vi "01 Dryer_Performance_SM.vi"() -> ()   [LabVIEW 2012] (continued)
                  tunnel: w1015 -> [w1034 _]
                  tunnel: [w1025 w1043] -> w1014
                  tunnel: [w1024 w1037] -> w1013
                  tunnel: w1012 -> [_ w1041]
                  tunnel: w1011 -> [_ w1040]
                  frame False {
                    n446 = call "AG34980A Initiate.vi"("VISA resource name"=w1036, "error in (no error)"=w1035) -> ("VISA resource name out"=w1032:refnum<visa-resource-name>, "error out"=w1033:errorcluster)  [unwired: 12 in]
                    n447 = call "AG34980A Fetch.vi"("VISA resource name"=w1032, "Numbers Only (T:On)"=TRUE, "error in (no error)"=w1033, "Byte Count (1024 bytes)"=5000) -> ("VISA resource name out"=w1021:refnum<visa-resource-name>, "Output Data (Numbers Only)"=w1027:dbl[], "error out"=w1023:errorcluster)  [unwired: 7 in, 2 out]
                    n448 = call "AG34980A Error Query (Multiple).vi"("VISA resource name"=w1021, "error in (no error)"=w1023) -> ("Error Message"=→"Error Message 2":string, "error out"=w1022:errorcluster)  [unwired: 10 in, 2 out]
                    n449 = Search 1D Array(1D array=w1034, element="Chamber Temp" ("Label")) -> (index of element=w1029:i32)  [unwired: 1 in]
                    n450 = Search 1D Array(1D array=w1034, element="Chamber RH" ("Label")) -> (index of element=w1030:i32)  [unwired: 1 in]
                    n451 = Index Array(array=w1027, index=w1029) -> (element=w1024:dbl)
                    n452 = Index Array(array=w1027, index=w1030) -> (element=w1025:dbl)
                  }
                  frame True {
                    n453 = local read "CDAQ Tasks"() -> (w1044:refnum<k21>[])
                    n454 = call "03 cDAQ Chan Tester.vi"("Tasks In"=w1044, "error in (no error)"=w1039, "Mode"=T18."Gather DATA") -> ("error out"=w1038:errorcluster, "CDAQ Data Out"=w1046:dbl[])  [unwired: 6 in, 1 out]
                    n455 = Decimal String To Number(string=w1041) -> (number=w1045:i32)  [unwired: 2 in, 1 out]
                    n456 = Decimal String To Number(string=w1040) -> (number=w1042:i32)  [unwired: 2 in, 1 out]
                    n457 = Index Array(array=w1046, index #1=w1045, index #2=w1042) -> (element #1=w1043:dbl, element #2=w1037:dbl)
                  }
                }
              }
              frame True {
                n458 = global read "Global Test Variables DPT.vi" "Globals for Dryer Performance Test"() -> (w1052:T9)
                n459 = Unbundle By Name(w1052) -> ("Test Setup.RH-IP"=w1053:string)
                n460 = call "Newport ITX-D3N.vi"("error in (no error)"=w1055, "Machine"=w1053) -> ("error out"=w1054:errorcluster, "[Temp (F), RH]"=w1051:dbl[])  [unwired: 8 in]
                n461 = Array To Cluster(array=w1051) -> (cluster=w1050:T26)
                n462 = Unbundle(w1050) -> ("[Temp (F), RH][0]"=w1049:dbl, "[Temp (F), RH][1]"=w1048:dbl)
              }
            }
            n463 = Number To Fractional String(number=w989, precision (6)=i16 1) -> (F-format string=w988:string)  [unwired: 2 in]
            n464 = Number To Fractional String(number=w986, precision (6)=i16 1) -> (F-format string=w985:string)  [unwired: 2 in]
            n465 = local read "2015?"() -> (w981:bool)
            n466 = Build Array("Ambient Temp", "Ambient RH") -> (w996:string[])
            n467 = Build Array(w985, w988) -> (w995:string[])
            n468 = Build Array(w996, w995) -> (w1004:string[][])
            n469 = call "Worksheet DOE Audit.vi"() -> ("DOE Data Out"=w991:T23)  [unwired: 8 in, 2 out]
            n470 = Bundle By Name(cluster=w991, "Ambinet Temp"=w985, "Ambinet RH"=w988) -> (w992:T23)
            n471 = Transpose 2D Array(2D array=w1004) -> (transposed array=w1003:string[][])
            n472 = Build Array (concatenate)(w1006, w1003) -> (w1005:string[][])
            n473 = Bundle By Name(cluster=w1008, "Start Header Data"=w1005) -> (w1007:T22)
            n474 = call "Worksheet DOE Audit.vi"("Add?"=TRUE, "DOE Data"=w992, "2015?"=w981) -> ()  [unwired: 5 in, 3 out]
          }
          frame True {
          }
        }
        n475 = case shown="Error" w972 {
          tunnel: ["" ("State(s) in Front (\"\")") "Macro: Exit" ("State(s) in Front (\"\")")] -> w978
          tunnel: w977 -> [_ w1060]
          frame No Error {
          }
          frame Error {
            n476 = Concatenate Strings("Error:", w1060) -> (w1062:string)
            n477 = One Button Dialog(message=w1062) -> ()  [unwired: 1 in, 1 out]
          }
        }
        n478 = call <vilib>:"Add State(s) to Queue__jki_lib_state_machine.vi"("State(s) in Front (\"\")"=w978, "State(s) in (\"\")"=w980) -> ("States Out"=w979:string)  [unwired: 13 in]
      }
      frame "Start: Files" {
        # "Preceeded by:\n Dryer Weight setting in Global."
        # "Alter File Init subvi per application to get a dialog box that gives you \nyour data filename."
        n479 = global read "Global Test Variables DPT.vi" "Globals for Dryer Performance Test"() -> (w1066:T9)
        n480 = local read "cDAQ"() -> (w1079:bool)
        n481 = Unbundle By Name(w1088) -> ("Start Header Data"=w1085:string[][])
        n482 = case shown="True" w1079 {
          frame False {
          }
          frame True {
            # "Keep CDAQ Buffer Empty"
            n483 = while {
              stop <- w1099 stop-if-true
              n484 = local read "CDAQ Tasks"() -> (w1100:refnum<k21>[])
              n485 = local read "Write to File"() -> (w1099:bool)
              n486 = call "03 cDAQ Chan Tester.vi"("Tasks In"=w1100, "Mode"=T18."Gather DATA") -> ()  [unwired: 7 in, 3 out]
              n487 = Wait (ms)(milliseconds to wait=u32 1000) -> ()  [unwired: 1 out]
            }
          }
        }
        n488 = Unbundle By Name(w1066) -> ("Directories.Work File Directory"=w1065:path)
        "Work File Directory" <- w1065
        n489 = local read "FileVersionInfo Out"() -> (w1080:T5)
        n490 = Unbundle By Name(w1080) -> ("ProductName"=w1095:string, "FileVersion"=w1094:string)
        n491 = local read "Scale Com Port"() -> (w1082:refnum<visa-resource-name>)
        n492 = call "Panel Data_File_Init DPT.vi"("Data File Directory"=w1065, "Test_Title Per TR:"="DPT" ("Test_Title*:"), "Scale Com Port"=w1082, "Test_Type:"=w1095, "Version In:"=w1094, "Supply Voltage:"="Supply Voltage:", "Flow Computer Info Baro,BTUF,u,Z"=w1085, "error in (no error)"=w1081, "File Extension:"="tmp") -> ("FileName"=w1068:path, "Nominal Load  Weight"=w1063:string, "Weights Out"=w1087:T27, "error out"=w1072:errorcluster)  [unwired: 2 in, 1 out]
        "FileName DataLog" <- w1068
        n493 = Bundle By Name(cluster=w1088, "Dryer Load Nominal Weight"=w1063) -> (w1064:T22)
        n494 = Strip Path(path=w1068) -> (name=w1078:string)  [unwired: 1 out]
        "Data Filename" <- w1078
        n495 = Match Pattern(string=w1078, regular expression="\\.") -> (before substring=w1076:string)  [unwired: 1 in, 3 out]
        n496 = Concatenate Strings(w1076, "_DC_AI.csv" ("string")) -> (w1073:string)
        n497 = Unbundle By Name(w1087) -> ("Actual RMC"=w1086:dbl, "Bone Dry Wt(lbs)"=w1084:dbl, "Measured IMC"=w1083:dbl)
        "BDW - Bone Dry Wt(lbs)" <- w1084
        "Wet Clothing Weight" <- w1083
        n498 = Build Path(base path=w1065, name or relative path=w1073) -> (appended path=w1074:path)
        n499 = local write "DC Voltages Filename"(w1074) -> ()
        n500 = Equal?(x=path "", y=w1068) -> (x = y?=w1067:bool)
        n501 = Unbundle By Name(w1072) -> ("status"=w1070:bool)
        n502 = flat-sequence {
          tunnel: w1084 -> [w1105]
          tunnel: w1083 -> [w1104]
          frame #0 {
            n503 = local read "2015?"() -> (w1102:bool)
            n504 = call "Worksheet DOE Audit.vi"() -> ("DOE Data Out"=w1107:T23)  [unwired: 8 in, 2 out]
            n505 = Bundle By Name(cluster=w1107, "Bone Dry Wt"=w1105, "Initial Wt"=w1104) -> (w1106:T23)
            n506 = call "Worksheet DOE Audit.vi"("Add?"=TRUE, "DOE Data"=w1106, "2015?"=w1102) -> ()  [unwired: 5 in, 3 out]
          }
        }
        n507 = local write "RMC%"(w1086) -> ()
        n508 = Or(x=w1067, y=w1070) -> (x .or. y?=w1071:bool)
        n509 = case shown="False" w1071 {
          tunnel: ["" ("State(s) in Front (\"\")") "Macro: Exit" ("State(s) in Front (\"\")")] -> w1089
          tunnel: w1090 -> [_ w1111]
          frame False {
            w1108 = TRUE
            n510 = property on="Write to File" class="Bool (strict)"("Val(Sgnl)"=w1108) -> ()  [unwired: 2 in, 2 out]
            "Write to File" <- w1108
          }
          frame True {
            n511 = Concatenate Strings("Error:", w1111) -> (w1113:string)
            n512 = One Button Dialog(message=w1113) -> ()  [unwired: 1 in, 1 out]
          }
        }
        n513 = call <vilib>:"Add State(s) to Queue__jki_lib_state_machine.vi"("State(s) in Front (\"\")"=w1089, "State(s) in (\"\")"=w1097) -> ("States Out"=w1096:string)  [unwired: 13 in]
      }
      frame "Get Offset Coeff" {
        # "w45 is the weight shift 45 seconds into the test.  The dryer scales have up to a 40 second averaging filter.\nAt 45 seconds after the dryer starts, take the weight adjusted for temp, and subtract from initial conditions.\nThis shift is correlated to the error at the end, depending on the load size."
        # "The conversion of weight to real weight:\n\nBase on load weight (first col).\nCoef of initial weight shift (second col.)\nOffset based on average error seen.  3rd col\nVolume used for temp calculations 4th col."
        n514 = global read "Global Test Variables DPT.vi" "Globals for Dryer Performance Test"() -> (w1116:T9)
        n515 = Unbundle By Name(w1133) -> ("Dryer Load Nominal Weight"=w1131:string)
        n516 = Decimal String To Number(string=w1131, default (0L)=0.0) -> (number=w1117:dbl)  [unwired: 1 in, 1 out]
        n517 = Unbundle By Name(w1116) -> ("Test Setup.T45_Coeff."=w1115:dbl, "Test Setup.Weight Offset"=w1114:dbl)
        n518 = In Range and Coerce(upper limit=3.0, x=w1117, lower limit=0.0) -> (In Range?=w1120:bool)  [unwired: 1 out]
        n519 = In Range and Coerce(upper limit=20.0, x=w1117, lower limit=4.0) -> (In Range?=w1122:bool)  [unwired: 1 out]
        n520 = In Range and Coerce(upper limit=4.0, x=w1117, lower limit=3.0) -> (In Range?=w1121:bool)  [unwired: 1 out]
        n521 = Build Array(w1120, w1121, w1122) -> (w1119:bool[])
        n522 = Boolean Array To Number(Boolean array=w1119) -> (number=w1118:u32)
        n523 = disable-structure shown="Disabled" {
          disable-tunnel: [w1139 w1147] -> w1134
          disable-tunnel: [w1138 w1146] -> w1129
          disable-tunnel: w1118 -> [w1137 _]
          disable-tunnel: w1115 -> [_ w1147]
          disable-tunnel: w1114 -> [_ w1146]
          frame Disabled {
            n524 = case shown="2" w1137 {
              tunnel: [0.0 ("Measured IMC") -1.3651 ("Measured IMC") -1.0373 ("Measured IMC")] -> w1139
              tunnel: [0.055 ("Offset") 0.0378 ("Offset") 0.0348 ("Offset")] -> w1138
              frame 0, Default {
              }
              frame 2 {
                # "4 lb load"
              }
              frame 1 {
              }
            }
          }
          frame Enabled {
          }
        }
        "Init Offset Coeff" <- w1134
        "Offset" <- w1129
        n525 = call <vilib>:"Add State(s) to Queue__jki_lib_state_machine.vi"("State(s) in (\"\")"=w1136) -> ("States Out"=w1135:string)  [unwired: 14 in]
      }
      frame "Start: Time" {
        # "Get stop condition.  Keep reading channels because cdaq gives error if buffer overflows."
        n526 = call "Panel Stop Condition.vi"() -> ("Enable Time Limit Out"=→"Enable Time Limit":bool, "Time Limit(s) Out"=→"Time Limit(s)":dbl, "Enable RMC Limit Out"=→"Enable RMC Limit":bool, "RMC Limit Out"=→"RMC Limit":dbl, "Enable Stop On Power Off Out"=→"Enable Stop On Power Off":bool, "Power Off Time(samples) Out"=→"Power Off Time(samples)":i32, "Power Off Check"=→"Power Off Check":bool[])  [unwired: 9 in]
        n527 = local read "cDAQ"() -> (w1148:bool)
        n528 = case shown="True" w1148 {
          frame False {
          }
          frame True {
            # "Keep CDAQ Buffer Empty"
            n529 = while {
              stop <- w1161 stop-if-true
              n530 = local read "CDAQ Tasks"() -> (w1162:refnum<k21>[])
              n531 = local read "Write to File"() -> (w1161:bool)
              n532 = call "03 cDAQ Chan Tester.vi"("Tasks In"=w1162, "Mode"=T18."Gather DATA") -> ()  [unwired: 7 in, 3 out]
              n533 = Wait (ms)(milliseconds to wait=u32 1000) -> ()  [unwired: 1 out]
            }
          }
        }
        n534 = call <vilib>:"Add State(s) to Queue__jki_lib_state_machine.vi"("State(s) in (\"\")"=w1159) -> ("States Out"=w1158:string)  [unwired: 14 in]
      }
      frame "---------- Data ----------" {
        # "Do not put any code in this frame.\n(It is a separator no-op. You can make a copy of this frame to create a new Data frame)"
        n535 = call <vilib>:"Add State(s) to Queue__jki_lib_state_machine.vi"("State(s) in (\"\")"=w1167) -> ("States Out"=w1166:string)  [unwired: 14 in]
      }
      frame "Data: Initialize" {
        w1168 = ""  # Dryer Load Nominal Weight
        w1169 = ""  # Dryer Type
        w1170 = string[][] []  # Start Header Data
        w1171 = 0.0  # Empty Dryer Cold Weight
        w1172 = "240/120"  # Supply Voltage:
        w1173 = string[] []  # DAQ Label List
        w1174 = ""  # DAQ Chan List
        w1175 = T6 {"Com Agilent"="COM1", "Com Flow Computer"="COM1", "Com Power Meter"="COM1", "Com Power Supply"=""}  # Equipment
        w1176 = path "C:/work/DryerPerformanceTest.ini"  # Config File Path
        w1177 = path "c:/palceholder.csv"  # FileName
        w1179 = errorcluster[] []  # Error Log
        w1180 = T28 {"Current VI Reference"=refnum, "Close Panel on Exit?"=FALSE}  # Core
        # "Config File Name"
        # "Initialize the shift-register data, here.\n(data names are defined by what you wire into the bundle function)"
        n536 = call <vilib>:"Add State(s) to Queue__jki_lib_state_machine.vi"("State(s) in (\"\")"=w1183) -> ("States Out"=w1182:string)  [unwired: 14 in]
        n537 = Bundle("Core"=w1180, "Error Log"=w1179, "FileName"=w1177, "Config File Path"=w1176, "Equipment"=w1175, "DAQ Chan List"=w1174, "DAQ Label List"=w1173, "Supply Voltage:"=w1172, "Empty Dryer Cold Weight"=w1171, "Start Header Data"=w1170, "Dryer Type"=w1169, "Dryer Load Nominal Weight"=w1168) -> (w1181:T22)  [unwired: 1 in]
      }
      frame "Data: Cleanup" {
        # "Cleanup any data and references, here.\n(this is called automatically, by the Macro: Exit)"
        n538 = Unbundle By Name(w1191) -> ("Core.Current VI Reference"=w1190:refnum<vi>, "Equipment.Com Flow Computer"=w1187:refnum<visa-resource-name>, "Equipment"=w1186:T6)
        n539 = flat-sequence {
          tunnel: w1190 -> [w1208]
          tunnel: w1189 -> [w1207]
          tunnel: [w1201] -> w1188
          tunnel: w1187 -> [w1206]
          tunnel: w1185 -> [w1204]
          tunnel: [w1202] -> w1184
          frame #0 {
            w1194 = TRUE ("Finish")
            n540 = Not(x=w1194) -> (.not. x?=w1195:bool)
            n541 = property on="End1_Main" class="Bool (strict)"("Val(Sgnl)"=w1194) -> ()  [unwired: 2 in, 2 out]
            n542 = global write "Nufi Global_ReceivedDataCluster.vi" "Exit Nufi"(w1194) -> ()
            n543 = local write "Start Test"(w1195) -> ()
            "End1_Main" <- w1194
          }
          frame #1 {
            n544 = while {
              stop <- w1200 stop-if-true
              n545 = local read "End2_DAQ"() -> (w1199:bool)
              n546 = local read "End4_Nufi"() -> (w1196:bool)
              n547 = local read "Eng3_Log"() -> (w1198:bool)
              n548 = Compound Arithmetic op=AND(w1196, w1199, w1198) -> (w1200:bool)
              n549 = Wait (ms)(milliseconds to wait=u32 150) -> ()  [unwired: 1 out]
            }
          }
          frame #2 {
            n550 = local read "Use SL9200 Gas Readings?"() -> (w1205:bool)
            n551 = for {
              tunnel: w1204 -> [w1212] mode=indexing
              n552 = VISA Close(VISA resource name=w1212) -> ()  [unwired: 1 in, 1 out]
            }
            n553 = case shown="False" w1205 {
              tunnel: w1206 -> [_ w1214]
              frame False {
              }
              frame True {
                n554 = call "SL9200_Driver_SM.vi"("ComPort"=w1214, "Close Com"=TRUE) -> ()  [unwired: 11 in, 3 out]
              }
            }
            n555 = Close Reference(reference=w1208, error in (no error)=w1207) -> (error out=w1203:errorcluster)
            n556 = case shown="Error" w1203 {
              selector: w1203 -> [w1209 w1210]
              tunnel: [_ "Exit" ("State(s) in Front (\"\")")] -> w1202
              tunnel: [w1209 _] -> w1201
              frame No Error {
              }
              frame Error {
                n557 = call <vilib>:"Simple Error Handler.vi"("error in (no error)"=w1210) -> ()  [unwired: 4 in, 5 out]
              }
            }
          }
        }
        n558 = Cluster To Array(cluster=w1186) -> (array=w1185:refnum<visa-resource-name>[])
        n559 = call <vilib>:"Add State(s) to Queue__jki_lib_state_machine.vi"("State(s) in Front (\"\")"=w1184, "State(s) in (\"\")"=w1193) -> ("States Out"=w1192:string)  [unwired: 13 in]
      }
      frame "---------- UI ----------" {
        # "Do not put any code in this frame.\n(It is a separator no-op. You can make a copy of this frame to create a new UI frame)"
        n560 = call <vilib>:"Add State(s) to Queue__jki_lib_state_machine.vi"("State(s) in (\"\")"=w1218) -> ("States Out"=w1217:string)  [unwired: 14 in]
      }
      frame "UI: Front Panel State" {
        # "Argument"
        # "Set Front Panel Open or Closed\n(Usage: \"UI: Front Panel State >> Open|Close|Minimize\")"
        n561 = Unbundle By Name(w1222) -> ("Core.Current VI Reference"=w1221:refnum<vi>)
        n562 = case shown="True" "Close when complete" {
          tunnel: w1224 -> [w1227 w1231]
          tunnel: [w1227 w1230] -> w1223
          tunnel: w1221 -> [_ w1229]
          tunnel: w1220 -> [_ w1228]
          frame False {
          }
          frame True {
            n563 = case shown="\"Close\"" w1228 {
              tunnel: w1231 -> [w1234 w1238 w1246]
              tunnel: [w1236 w1241 w1247] -> w1230
              tunnel: w1229 -> [w1235 w1237 w1244]
              frame "Open", Default {
                n564 = invoke class="VI" method="FP.Open"(reference=w1235, error in=w1234, "Activate"=TRUE, "State"=T21."Maximized") -> (error out=w1236:errorcluster)  [unwired: 1 in, 4 out]
              }
              frame "Minimize" {
                n565 = invoke class="VI" method="FP.Open"(reference=w1237, error in=w1238, "Activate"=TRUE, "State"=T21."Minimized") -> (error out=w1241:errorcluster)  [unwired: 1 in, 4 out]
              }
              frame "Close" {
                n566 = property class="VI"(reference=w1244, error in=w1246) -> (reference out=w1243:refnum<vi>, error out=w1245:errorcluster, "Front Panel.Open"=w1242:bool)
                n567 = case shown="True" w1242 {
                  tunnel: [w1248 w1251] -> w1247
                  tunnel: w1245 -> [w1248 w1250]
                  tunnel: w1243 -> [_ w1249]
                  frame False {
                  }
                  frame True {
                    n568 = invoke class="VI" method="FP.Close"(reference=w1249, error in=w1250) -> (error out=w1251:errorcluster)  [unwired: 1 in, 2 out]
                  }
                }
              }
            }
          }
        }
        n569 = call <vilib>:"Add State(s) to Queue__jki_lib_state_machine.vi"("State(s) in (\"\")"=w1226) -> ("States Out"=w1225:string)  [unwired: 14 in]
      }
      frame "-------Config File------" {
        # "Do not put any code in this frame.\n(It is a separator no-op. You can make a copy of this frame to create a new Data frame)"
        n570 = call <vilib>:"Add State(s) to Queue__jki_lib_state_machine.vi"("State(s) in (\"\")"=w1255) -> ("States Out"=w1254:string)  [unwired: 14 in]
      }
      frame "Config: Read" {
        w1264 = FALSE  # Write?
        # "Read Globals from Config File.\n(This file will be customized per application)"
        n571 = Unbundle By Name(w1267) -> ("Config File Path"=w1263:path)
        n572 = call "Global Cluster ReadWrite.vi"("Write?"=w1264, "error in (no error)"=w1266, "configuration file path"=w1263) -> ("error out"=w1265:errorcluster, "Test Config Out"=w1257:T9)  [unwired: 7 in]
        n573 = global write "Global Test Variables DPT.vi" "Globals for Dryer Performance Test"(w1257) -> ()
        n574 = local write "Globals for Dryer Performance Test"(w1257) -> ()
        n575 = Unbundle By Name(w1257) -> ("Test Setup.Scale Com"=w1262:dbl, "Test Setup.W. Samps"=w1259:i32, "Test Setup.Smoothing"=→"Use Smoothing":bool, "Test Setup.CDAQ"=→"cDAQ":bool)
        n576 = To Unsigned Byte Integer(number=w1262) -> (unsigned 8bit integer=w1261:u8)
        n577 = call "Com Chan Type Conversion.vi"("Com Chan"=w1261) -> ("VISA resource name"=→"Scale Com Port":refnum<visa-resource-name>)  [unwired: 11 in, 3 out]
        n578 = call <vilib>:"Add State(s) to Queue__jki_lib_state_machine.vi"("State(s) in (\"\")"=w1269) -> ("States Out"=w1268:string)  [unwired: 14 in]
        n579 = local write "W.Samps"(w1259) -> ()
      }
      frame "Config: Write" {
        # "Write Globals to Config File.\n(This file will be customized per application)"
        n580 = Unbundle By Name(w1275) -> ("Config File Path"=w1274:path)
        n581 = global read "Global Test Variables DPT.vi" "Globals for Dryer Performance Test"() -> (w1270:T9)
        "Globals for Dryer Performance Test" <- w1270
        n582 = call "Global Cluster ReadWrite.vi"("Write?"=TRUE, "error in (no error)"=w1273, "configuration file path"=w1274, "Test Config In"=w1270) -> ("error out"=w1272:errorcluster)  [unwired: 6 in, 1 out]
        n583 = call <vilib>:"Add State(s) to Queue__jki_lib_state_machine.vi"("State(s) in (\"\")"=w1277) -> ("States Out"=w1276:string)  [unwired: 14 in]
      }
      frame "---------- Macro ----------" {
        # "Do not put any code in this frame.\n(It is a separator no-op. You can make a copy of this frame to create a new Macro frame)"
        n584 = call <vilib>:"Add State(s) to Queue__jki_lib_state_machine.vi"("State(s) in (\"\")"=w1281) -> ("States Out"=w1280:string)  [unwired: 14 in]
      }
      frame "Macro: Initialize" {
        # "Initialization Macro\n(This is called once, when the VI starts)"
        n585 = call <vilib>:"Add State(s) to Queue__jki_lib_state_machine.vi"("State(s) in Front (\"\")"="Data: Initialize\nInitialize Core Data\nUI: Front Panel State >> Minimize", "State(s) in (\"\")"=w1286) -> ("States Out"=w1285:string)  [unwired: 13 in]
      }
      frame "Macro: Exit" {
        w1296 = "\n"
        w1298 = "Stopping Test" ("String")
        # "Exit Macro\n(This is called once, when the VI exits)"
        n586 = Unbundle By Name(w1300) -> ("Core.Close Panel on Exit?"=w1292:bool)
        n587 = local read "exe?"() -> (w1291:bool)
        n588 = call "String_in_Reference.vi"("String"=w1298) -> ()  [unwired: 18 in, 1 out]
        n589 = local write "Status Message"(w1298) -> ()
        n590 = Compound Arithmetic op=AND(w1292, w1291) -> ()  [unwired: 1 out]
        n591 = Select(t="UI: Front Panel State >> Close", s=FALSE, f="") -> (s? t:f=w1295:string)
        n592 = local write "End Test Button"(FALSE ("End Test")) -> ()
        n593 = Concatenate Strings("Data: Cleanup", w1296, w1295, w1296, "Exit") -> (w1293:string)
        n594 = property on="stop" class="Bool (strict)"("Val(Sgnl)"=TRUE ("Value (Signaling)")) -> ()  [unwired: 2 in, 2 out]
        n595 = call <vilib>:"Add State(s) to Queue__jki_lib_state_machine.vi"("State(s) in Front (\"\")"=w1293, "State(s) in (\"\")"=w1303) -> ("States Out"=w1302:string)  [unwired: 13 in]
      }
      frame "---------- Test ----------" {
        n596 = call <vilib>:"Add State(s) to Queue__jki_lib_state_machine.vi"("State(s) in (\"\")"=w1307) -> ("States Out"=w1306:string)  [unwired: 14 in]
      }
      frame "Test: Main" {
        # "Wait for the test to complete.  Either the button is pressed, or RMC limit is reached, or the time is reached, or the power is off."
        # "Use this as a test to see if the test is complete.  If not, continue to wait."
        n597 = local read "Enable Stop On Power Off"() -> (w1308:bool)
        n598 = local read "Power Off Time(samples)"() -> (w1316:i32)
        n599 = local read "Enable Time Limit"() -> (w1309:bool)
        n600 = local read "Power On One Shot"() -> (w1311:bool)
        n601 = local read "Enable RMC Limit"() -> (w1310:bool)
        n602 = local write "Loggin Data"(TRUE ("Init Complete")) -> ()
        n603 = call "String_in_Reference.vi"("String"="Running, Logging Data...") -> ()  [unwired: 18 in, 1 out]
        n604 = And(x=w1308, y=w1311) -> (x .and. y?=w1317:bool)
        n605 = And(x=w1310, y=w1311) -> (x .and. y?=w1312:bool)
        n606 = case shown="True" w1309 {
          tunnel: [FALSE w1350] -> w1322
          frame False {
          }
          frame True {
            n607 = local read "Start Time (sec)"() -> (w1349:dbl)
            n608 = local read "Time Limit(s)"() -> (w1346:dbl)
            n609 = call "E-Time.vi"() -> ("Elapsed Time (sec)"=w1348:dbl)  [unwired: 9 in, 2 out]
            n610 = Subtract(x=w1348, y=w1349) -> (x-y=w1347:dbl)
            n611 = Greater?(x=w1347, y=w1346) -> (0:w1350:bool)
          }
        }
        n612 = case shown="True" w1312 {
          tunnel: [FALSE w1344] -> w1315
          frame False {
          }
          frame True {
            n613 = local read "RMC Limit"() -> (w1342:dbl)
            n614 = local read "RMC%"() -> (w1343:dbl)
            n615 = Greater?(x=w1342, y=w1343) -> (0:w1344:bool)
          }
        }
        n616 = case shown="True" w1317 {
          selector: w1317 -> [w1329 _]
          tunnel: w1316 -> [_ w1331]
          tunnel: [w1329 w1330] -> w1314
          frame False {
          }
          frame True {
            n617 = disable-structure shown="Enabled" {
              disable-tunnel: w1331 -> [w1338 _]
              disable-tunnel: [w1332 w1340] -> w1330
              frame Disabled {
                n618 = call "Counter.vi"() -> ("Count"=w1339:dbl)  [unwired: 11 in]
                n619 = local read "Power Off Check"() -> (w1335:bool[])
                n620 = Quotient & Remainder(x=w1339, y=w1338) -> (x-y*floor(x/y)=w1337:dbl)  [unwired: 1 out]
                n621 = local read "Power On"() -> (w1336:bool)
                n622 = Replace Array Subset(array=w1335, new element=w1336, index=w1337) -> (w1334:bool[])
                n623 = local write "Power Off Check"(w1334) -> ()
                n624 = Not(x=w1334) -> (.not. x?=w1333:bool[])
                n625 = And Array Elements(Boolean array=w1333) -> (logical AND=w1332:bool)
              }
              frame Enabled {
                n626 = local read "Power Off One Shot"() -> (w1340:bool)
              }
            }
          }
        }
        n627 = local read "End Test Button"() -> (w1313:bool)
        n628 = Compound Arithmetic op=OR(w1322, w1315, w1313, w1314) -> (w1321:bool)
        "Test Complete?" <- w1321
        n629 = case shown="True" w1321 {
          tunnel: ["Test: Control Sequence" ("State(s) at Back (\"\")") "Power Off\nMacro: Exit" ("State(s) in Front (\"\")")] -> w1325
          tunnel: w1315 -> [_ w1355]
          tunnel: w1314 -> [_ w1354]
          tunnel: w1313 -> [_ w1353]
          frame False {
          }
          frame True {
            n630 = case shown="False" w1355 {
              tunnel: w1354 -> [_ w1366]
              tunnel: [w1357 w1365] -> w1352
              tunnel: w1353 -> [_ w1364]
              frame True {
                n631 = local read "Start Time (sec)"() -> (w1362:dbl)
                n632 = call "E-Time.vi"() -> ("Elapsed Time (sec)"=w1363:dbl)  [unwired: 9 in, 2 out]
                n633 = Subtract(x=w1363, y=w1362) -> (x-y=w1361:dbl)
                n634 = Number To Fractional String(number=w1361) -> (F-format string=w1360:string)  [unwired: 3 in]
                n635 = Concatenate Strings("RMC Limit Reached: Cycle Time, ", w1360, ", seconds.") -> (w1357:string)
              }
              frame False {
                n636 = case shown="True" w1366 {
                  tunnel: [w1367 w1376] -> w1365
                  tunnel: w1364 -> [w1368 _]
                  frame False {
                    n637 = Select(t="End Button Depressed", s=w1368, f="Over Time Limit") -> (s? t:f=w1367:string)
                  }
                  frame True {
                    n638 = local read "Start Time (sec)"() -> (w1381:dbl)
                    n639 = local read "2015?"() -> (w1371:bool)
                    n640 = local read "Tend?"() -> (w1372:dbl)
                    n641 = Subtract(x=w1372, y=w1381) -> (x-y=w1380:dbl)
                    n642 = Number To Fractional String(number=w1380) -> (F-format string=w1379:string)  [unwired: 3 in]
                    n643 = call "Worksheet DOE Audit.vi"() -> ("DOE Data Out"=w1374:T23)  [unwired: 8 in, 2 out]
                    n644 = Bundle By Name(cluster=w1374, "End Time(s)"=w1372) -> (w1373:T23)
                    n645 = Concatenate Strings("Power Off: Cycle Time, ", w1379, ", seconds.") -> (w1376:string)
                    n646 = call "Worksheet DOE Audit.vi"("Add?"=TRUE, "DOE Data"=w1373, "2015?"=w1371) -> ()  [unwired: 5 in, 3 out]
                  }
                }
              }
            }
            "End Msg" <- w1352
          }
        }
        n647 = local read "UI Timer"() -> (w1320:i32)
        n648 = To Unsigned Long Integer(number=w1320) -> (unsigned 32bit integer=w1319:u32)
        n649 = Wait (ms)(milliseconds to wait=w1319) -> ()  [unwired: 1 out]
        n650 = call <vilib>:"Add State(s) to Queue__jki_lib_state_machine.vi"("State(s) in Front (\"\")"=w1325, "State(s) in (\"\")"=w1328) -> ("States Out"=w1327:string)  [unwired: 13 in]
      }
      frame "Test: Control Sequence" {
        # "Main control sequence defined here."
        n651 = call <vilib>:"Add State(s) to Queue__jki_lib_state_machine.vi"("State(s) in Front (\"\")"="Test: Step 1" ("State(s) in Front (\"\")"), "State(s) in (\"\")"=w1386) -> ("States Out"=w1385:string)  [unwired: 13 in]
      }
      frame "Test: Step 1" {
        # "Description of Test Step.\nCheck Every Minute if you are done."
        n652 = call <vilib>:"Add State(s) to Queue__jki_lib_state_machine.vi"("State(s) in Front (\"\")"="Test: Main" ("State(s) in Front (\"\")"), "State(s) in (\"\")"=w1391) -> ("States Out"=w1390:string)  [unwired: 13 in]
      }
      frame "-----Functions------" {
        n653 = call <vilib>:"Add State(s) to Queue__jki_lib_state_machine.vi"("State(s) in (\"\")"=w1395) -> ("States Out"=w1394:string)  [unwired: 14 in]
      }
      frame "Power Off" {
        n654 = local read "Simulate"() -> (w1400:bool)
        n655 = Unbundle By Name(w1402) -> ("Equipment.Com Power Supply"=w1401:refnum<visa-resource-name>)
        n656 = case shown="False" w1400 {
          tunnel: w1401 -> [w1413 _]
          tunnel: [w1411 w1419] -> w1398
          tunnel: w1399 -> [w1412 w1419]
          frame False {
            n657 = local read "Use Chroma"() -> (w1410:bool)
            n658 = case shown="False" w1410 {
              tunnel: w1413 -> [_ w1418]
              tunnel: w1412 -> [w1414 w1417]
              tunnel: [w1414 w1416] -> w1411
              frame False {
              }
              frame True {
                n659 = call "Chroma Driver GPIB-VISA-RW.vi"("VISA resource name"=w1418, "Chroma Power Select"=Chroma_Driver_Select."Output Off", "error in (no error)"=w1417) -> ("error out"=w1416:errorcluster)  [unwired: 11 in, 1 out]
              }
            }
          }
          frame True {
          }
        }
        n660 = case shown="Error" w1398 {
          tunnel: ["" ("State(s) in Front (\"\")") "Macro: Exit" ("State(s) in Front (\"\")")] -> w1397
          tunnel: w1396 -> [_ w1407]
          frame No Error {
          }
          frame Error {
            n661 = Concatenate Strings("Error:", w1407) -> (w1409:string)
            n662 = One Button Dialog(message=w1409) -> ()  [unwired: 1 in, 1 out]
          }
        }
        n663 = call <vilib>:"Add State(s) to Queue__jki_lib_state_machine.vi"("State(s) in Front (\"\")"=w1397, "State(s) in (\"\")"=w1404) -> ("States Out"=w1403:string)  [unwired: 13 in]
      }
    }
    n664 = local read "Debug Mode"() -> (w61:bool)
    n665 = case shown="True" w61 {
      tunnel: [w75 w78] -> w65
      tunnel: w64 -> [w75 w77]
      tunnel: w62 -> [_ w76]
      frame False {
      }
      frame True {
        n666 = Build Array (concatenate)(w77, w76) -> (w78:string[])
        "Debug List Test States" <- w78
      }
    }
  }
  "error out" <- w10
  n667 = call <vilib>:"Add State(s) to Queue__jki_lib_state_machine.vi"("State(s) in (\"\")"="Data: Initialize") -> ("States Out"=w14:string)  [unwired: 14 in]
  n668 = while "Data Procressing, UI Update, Data Storage" {
    shift-right: [w1429] -> _
    shift-left: _ -> [w1428]
    shift-right: [w1431] -> _
    shift-left: _ -> [w1427]
    shift-right: [w1430] -> _
    shift-left: w4 -> [w1432]
    tunnel: w23 -> [w1426]
    shift-right: [w1424] -> w21
    shift-left: string[] [] -> [w1425]
    tunnel: [w1420] -> w26
    stop <- w1420 stop-if-true
    n669 = call <vilib>:"Parse State Queue__jki_lib_state_machine.vi"("State Queue"=w1432, "Error In (no error)"=w1427) -> ("Remaining States"=w1434:string, "Current State"=w1423:string, "Arguments"=w1433:string)  [unwired: 11 in]
    n670 = case shown="\"Finalize DataLog\"" w1423 {
      selector: w1423 -> [_ w1479 _ _ _ _ _ _ _ _ _ _ _ _ _ _ _ _ _ _ _ _ _ _ _]
      tunnel: w1434 -> [w1445 w1483 w1495 w1499 w1507 w1513 w1521 w1536 w1553 w1579 w1619 w1691 w1722 w1756 w1768 w1859 w1905 w1946 w1956 w1965 w2020 w2050 w2082 w2154 w2191]
      tunnel: w1433 -> [_ _ _ _ _ w1509 _ _ _ _ _ _ _ _ _ _ _ _ _ _ _ _ _ _ _]
      tunnel: w1428 -> [w1443 w1481 w1492 w1496 w1504 w1508 w1518 w1533 w1550 w1572 w1613 w1689 w1716 w1753 w1762 w1854 w1900 w1942 w1953 w1962 w2017 w2047 w2079 w2151 w2187]
      tunnel: [w1442 w1485 errorcluster {"status"=FALSE, "code"=0, "source"=""} ("error out") w1497 w1505 w1511 w1519 w1534 w1551 w1577 w1617 w1635 w1711 w1754 w1766 w1857 w1903 w1944 w1954 w1963 w2018 w2048 w2080 w2129 w2189] -> w1431
      tunnel: w1427 -> [w1441 w1484 w1491 w1497 w1505 w1510 w1519 w1534 w1551 w1577 w1617 w1635 w1712 w1754 w1766 w1857 w1903 w1944 w1954 w1963 w2018 w2048 w2080 w2124 w2189]
      tunnel: [w1444 w1482 w1494 w1498 w1506 w1512 w1520 w1535 w1552 w1578 w1618 w1690 w1721 w1755 w1767 w1858 w1904 w1945 w1955 w1964 w2019 w2049 w2081 w2153 w2190] -> w1430
      tunnel: [_ _ _ _ _ _ _ _ _ _ _ _ _ _ _ _ _ _ _ _ _ _ _ TRUE TRUE] -> w1420
      tunnel: [w1440 w1481 w1492 w1496 w1504 w1508 w1518 w1532 w1549 w1571 w1613 w1688 w1715 w1753 w1765 w1855 w1900 w1942 w1953 w1962 w2017 w2047 w2079 w2151 w2187] -> w1429
      tunnel: "UI Timer" -> [w1439 _ _ _ _ _ _ _ _ _ _ _ _ _ _ _ _ _ _ _ _ _ _ _ _]
      tunnel: w1426 -> [_ _ _ _ _ _ _ w1531 w1548 _ _ _ _ _ _ _ _ _ _ _ _ _ _ _ _]
      frame "", "Idle" {
        # "executes when the state queue is empty"
        n671 = event shown="[0] Timeout" {
          selector: _ -> [_ _ _]
          dyn-events: _ -> [_ _ _]
          timeout: w1439 -> [_ _ _]
          tunnel: w1445 -> [w1450 _ _]
          tunnel: [w1449 w1453 w1466] -> w1444
          tunnel: w1443 -> [w1447 w1454 w1463]
          tunnel: [w1448 w1451 w1464] -> w1442
          tunnel: w1441 -> [w1448 w1451 w1464]
          tunnel: [w1447 w1454 w1463] -> w1440
          event Timeout {
            n672 = event-data() -> ()  [unwired: 1 in, 1 out]
            n673 = call <vilib>:"Add State(s) to Queue__jki_lib_state_machine.vi"("State(s) in Front (\"\")"="UI: Update", "State(s) in (\"\")"=w1450) -> ("States Out"=w1449:string)  [unwired: 13 in]
          }
          event "# elements in queue": Value Change {
            n674 = event-data() -> ()  [unwired: 1 in, 6 out]
            n675 = call <vilib>:"Add State(s) to Queue__jki_lib_state_machine.vi"("State(s) in Front (\"\")"="Data: DeQueue\nData: Process\nData: Save\nUI: Update" ("State(s) in Front (\"\")")) -> ("States Out"=w1453:string)  [unwired: 14 in]
          }
          event "End1_Main": Value Change {
            n676 = event-data() -> ()  [unwired: 1 in, 6 out]
            n677 = Unbundle By Name(w1463) -> ("Q Element.Label Array"=w1460:string[], "Q Element.Data Array"=w1459:dbl[])
            n678 = local read "Use Dry Gas Meter?"() -> (w1457:bool)
            n679 = local read "Write to File"() -> (w1455:bool)
            n680 = Search 1D Array(1D array=w1460, element="Gas Feedback") -> (index of element=w1462:i32)  [unwired: 1 in]
            n681 = And(x=w1457, y=w1455) -> (x .and. y?=w1456:bool)
            n682 = Index Array(array=w1459, index=w1462) -> (element=w1458:dbl)
            n683 = case shown="True" w1456 {
              tunnel: w1458 -> [_ w1470]
              frame False {
              }
              frame True {
                n684 = Number To Fractional String(number=w1470, precision (6)=i16 3) -> (F-format string=w1469:string)  [unwired: 2 in]
                n685 = Fract/Exp String To Number(string=w1469) -> (number=w1471:dbl)  [unwired: 3 in, 1 out]
                n686 = call "Worksheet DOE Audit.vi"() -> ("DOE Data Out"=w1472:T23)  [unwired: 8 in, 2 out]
                n687 = local read "2015?"() -> (w1467:bool)
                n688 = Bundle By Name(cluster=w1472, "Gas Vol Fin"=w1471) -> (w1473:T23)
                n689 = Concatenate Strings("Dry Meter Final Reading", "," ("string"), w1469) -> (w1477:string)
                n690 = local read "FileName DataLog"() -> (w1476:path)
                n691 = call "Log String to Spreadsheet.vi"("String"=w1477, "FileName"=w1476) -> ()  [unwired: 9 in, 1 out]
                n692 = call "Worksheet DOE Audit.vi"("Add?"=TRUE, "DOE Data"=w1473, "2015?"=w1467) -> ()  [unwired: 5 in, 3 out]
              }
            }
            n693 = call <vilib>:"Add State(s) to Queue__jki_lib_state_machine.vi"("State(s) in Front (\"\")"="Finalize Sequence\nExit" ("State(s) in Front (\"\")")) -> ("States Out"=w1466:string)  [unwired: 14 in]
          }
        }
      }
      frame Default {
        w1488 = 42 items=["No error", "Argument error", "Memory is full", "Out of zone", "End of file", "File already open", "Generic file I/O error", "File not found", "File permission error", "Disk is full", "Duplicate path", "Too many files open", "System feature not enabled", "Resource file not found", "Cannot add resource", "Resource not found", "Image not found", "Image memory error", "Pen does not exist", "Config type invalid", "Config token not found", "Config parse error", "Config memory error", "Bad external code format", "Bad external code offset", "External code not present", "Null window", "Destroy window error", "Null menu", "Print aborted", "Bad print record", "Print driver error", "Windows error during printing", "Memory error during printing", "Print dialog error", "Generic print error", "Invalid device refnum", "Device not found", "Device parameter error", "Device unit error", "Cannot open device", "Device call aborted", "Generic error", "Cancelled by user", "Object ID too low", "Object ID too high", "Object not in heap", "Unknown heap", "Unknown object (invalid DefProc)", "Unknown object (DefProc not in table)", "Message out of range", "Invalid (null) method", "Unknown message", "Manager call not supported", "Bad address", "Network operation in progress", "Network operation timed out", "Connection is busy", "Network attribute not supported", "Network error", "Address in use", "System out of memory", "Connection aborted", "Connection refused", "Not connected", "Already connected", "Connection closed", "Initialization error (interapplication manager)", "Bad occurrence", "Wait on unbound occurrence handler", "Occurrence queue overflow", "Datalog type conflict", "Unused", "Unrecognized type (interapplication manager)", "Memory corrupt", "Failed to make temporary DLL", "Old CIN version", "Drag socket not found", "Failed to load drop-object", "Failed to register OLE object", "Failed to release OLE object", "Format specifier type mismatch", "Unknown format specifier", "Too few format specifiers", "Too many format specifiers", "Scan failed", "Newer CIN version", "Error converting to variant", "Runtime menu error", "Password tampered", "Variant attribute not found", "Incompatible variant data type", "Event data is not available", "Event Store is not present", "Occurrence is not found", "Event Queue is not created", "Event info is not available", "Refnum passed is NULL", "Error retrieving Class GUID", "Error retrieving CoClass GUID", "Error retrieving TypeLib GUID.", "Bad built application magic bytes.", "Specific driver is different from the specific driver associated with the Logical Name.", "There is no session opened to the class driver.", "Max Error", "MAX - Error with config objects", "MAX - Error loading configuration", "MAX - Group not supported"]
        # "Current State"
        # "Do not delete, rename, or modify this frame.\n(this is used to capture unhandled states and typos)"
        # "Handle mistyped state name (developer tool)"
        n694 = Format Into String(format string="Software Exception: Unhandled State \"%s\"." ("message"), error in=w1484, w1479) -> (resulting string=w1487:string, error out=w1486:errorcluster)  [unwired: 1 in]
        n695 = call <vilib>:"Error Cluster From Error Code.vi"("show call chain? (False)"=TRUE, "error in (no error)"=w1486, "error message (\"\")"=w1487, "error code (0)"=w1488) -> ("error out"=w1485:errorcluster)  [unwired: 5 in]
        n696 = call <vilib>:"Add State(s) to Queue__jki_lib_state_machine.vi"("State(s) in (\"\")"=w1483) -> ("States Out"=w1482:string)  [unwired: 14 in]
      }
      frame "Error Handler" {
        # "Unhandled Error -- Display it"
        # "Handle any errors here.\nYou can also output any states to clean-up after errors occur"
        # "Clear error"
        n697 = call <vilib>:"General Error Handler.vi"("error in (no error)"=w1491) -> ()  [unwired: 10 in, 5 out]
        n698 = call <vilib>:"Add State(s) to Queue__jki_lib_state_machine.vi"("State(s) in Front (\"\")"="/* Post Error States", "State(s) in (\"\")"=w1495) -> ("States Out"=w1494:string)  [unwired: 13 in]
      }
      frame "---------- UI ----------" {
        # "Do not put any code in this frame.\n(It is a separator no-op. You can make a copy of this frame to create a new Data frame)"
        n699 = call <vilib>:"Add State(s) to Queue__jki_lib_state_machine.vi"("State(s) in (\"\")"=w1499) -> ("States Out"=w1498:string)  [unwired: 14 in]
      }
      frame "UI: Update" {
        # "Update User Interface with processed Data"
        n700 = local read "Start Time (sec)"() -> (w1501:dbl)
        n701 = call "E-Time.vi"() -> ("Elapsed Time (sec)"=w1500:dbl)  [unwired: 9 in, 2 out]
        n702 = call "String_in_Reference.vi"() -> ("String Out"=→"Status Message":string)  [unwired: 19 in]
        n703 = Subtract(x=w1500, y=w1501) -> (x-y=→"Elapsed Time":dbl)
        n704 = call <vilib>:"Add State(s) to Queue__jki_lib_state_machine.vi"("State(s) in (\"\")"=w1507) -> ("States Out"=w1506:string)  [unwired: 14 in]
      }
      frame "UI: Cursor Set" {
        # "Argument"
        # "Set and Unset Cursor Busy.\n(Usage: \"UI: Cursor Set >> Busy|Idle\")"
        n705 = case shown="\"Idle\", Default" w1509 {
          tunnel: w1510 -> [w1515 w1517]
          tunnel: [w1514 w1516] -> w1511
          frame "Idle", Default {
            n706 = call <vilib>:"Unset Busy.vi"("error in (no error)"=w1515) -> ("error out"=w1514:errorcluster)  [unwired: 10 in]
          }
          frame "Busy" {
            n707 = call <vilib>:"Set Busy.vi"("error in (no error)"=w1517) -> ("error out"=w1516:errorcluster)  [unwired: 9 in, 1 out]
          }
        }
        n708 = call <vilib>:"Add State(s) to Queue__jki_lib_state_machine.vi"("State(s) in (\"\")"=w1513) -> ("States Out"=w1512:string)  [unwired: 14 in]
      }
      frame "------ DATA ------" {
        # "Do not put any code in this frame.\n(It is a separator no-op. You can make a copy of this frame to create a new Data frame)"
        n709 = call <vilib>:"Add State(s) to Queue__jki_lib_state_machine.vi"("State(s) in (\"\")"=w1521) -> ("States Out"=w1520:string)  [unwired: 14 in]
      }
      frame "Data: Initialize" {
        w1524 = FALSE  # Power Previous
        w1525 = FALSE  # Enable RMC
        w1528 = dbl[] []  # Time Array
        w1527 = dbl[][] []  # Data Array
        w1526 = TRUE  # Init Save File
        w1529 = TRUE  # Graph Reset
        # "Offset value init."
        n710 = call "FGV Double.vi"("Value In"=0.0, "Set?"=TRUE) -> ()  [unwired: 9 in, 1 out]
        n711 = local read "Q Element"() -> (w1530:T10)
        n712 = call <vilib>:"Add State(s) to Queue__jki_lib_state_machine.vi"("State(s) in (\"\")"=w1536) -> ("States Out"=w1535:string)  [unwired: 14 in]
        n713 = Bundle(cluster=w1533, "queue out"=w1531, "Q Element"=w1530, "Graph Reset"=w1529, "Init Save File"=w1526, "Time Array"=w1528, "Data Array"=w1527, "Enable RMC"=w1525, "Power Previous"=w1524) -> (w1532:T29)
      }
      frame "Data: DeQueue" {
        # "Remove Time"
        # "Your code here.\n(You can make a copy of, or modify, this frame)"
        n714 = Dequeue Element(queue=w1548) -> (element=w1547:T10)  [unwired: 2 in, 3 out]
        n715 = Unbundle By Name(w1547) -> ("Label Array"=w1545:string[], "Data Array"=w1540:dbl[])
        n716 = local read "Plot Legend"() -> (w1542:T2)
        n717 = Number To Fractional String(number=w1540) -> (F-format string=w1546:string[])  [unwired: 3 in]
        n718 = Delete From Array(array=w1540, length=1, index=0) -> (array with subset deleted=w1539:dbl[])  [unwired: 1 out]
        n719 = Build Array(w1545, w1546) -> (w1544:string[][])
        n720 = for {
          tunnel: w1539 -> [w1555] mode=indexing
          tunnel: w1542 -> [w1556] mode=indexing
          tunnel: [w1554] -> w1541 mode=indexing
          n721 = Bundle By Name(cluster=w1556, "Value"=w1555) -> (w1554:T30)
        }
        n722 = Transpose 2D Array(2D array=w1544) -> (transposed array=→"Data":string[][])
        n723 = Bundle By Name(cluster=w1550, "Q Element"=w1547) -> (w1549:T29)
        n724 = local write "Plot Legend"(w1541) -> ()
        n725 = call <vilib>:"Add State(s) to Queue__jki_lib_state_machine.vi"("State(s) in (\"\")"=w1553) -> ("States Out"=w1552:string)  [unwired: 14 in]
      }
      frame "Data: Process" {
        # "Disable RMC during power off."
        # "If the current indicates the the dryer is on, go to the Data: Process RMC"
        n726 = Unbundle By Name(w1572) -> ("Q Element.Label Array"=w1565:string[], "Q Element.Data Array"=w1564:dbl[], "Enable RMC"=w1570:bool)
        n727 = local read "Write to File"() -> (w1557:bool)
        n728 = Search 1D Array(1D array=w1565, element="P:Sigma") -> (index of element=w1567:i32)  [unwired: 1 in]
        n729 = Index Array(array=w1564, index=w1567) -> (element=w1575:dbl)
        n730 = Greater?(x=w1575, y="Power On Threshold") -> (0:w1558:bool)
        n731 = And(x=w1558, y=w1557) -> (x .and. y?=w1559:bool)
        "Power On" <- w1559
        n732 = call "Dryer Power Latches.vi"("Time Limit in Seconds"="Power off Check RMC sec", "Power On"=w1559) -> ("Time of Last Power On"=w1561:dbl, "Power Off One Shot"=w1562:bool, "Power On One Shot"=w1563:bool)  [unwired: 7 in]
        "Power On One Shot" <- w1563
        "Power Off One Shot" <- w1562
        n733 = Compound Arithmetic op=AND(w1563, invert w1562, w1557) -> (w1568:bool)
        n734 = Compound Arithmetic op=AND(w1568, invert w1570) -> (w1569:bool)
        n735 = case shown="True" w1569 {
          tunnel: w1565 -> [_ w1596]
          tunnel: w1564 -> [_ w1595]
          tunnel: string[] ["Wp:Sigma", "Tscale", "Gas Pressure", "Gas Temperature", "Barometric Pressure", "Gas Feedback"] ("Label List 2") -> [_ w1597]
          frame False {
          }
          frame True {
            # "First time through, init. start time."
            n736 = for {
              tunnel: w1595 -> [w1610]
              tunnel: w1596 -> [w1609]
              tunnel: w1597 -> [w1608] mode=indexing
              tunnel: [w1607] -> w1594 mode=indexing
              n737 = Search 1D Array(1D array=w1609, element=w1608) -> (index of element=w1611:i32)  [unwired: 1 in]
              n738 = Index Array(array=w1610, index=w1611) -> (element=w1607:dbl)
            }
            n739 = local read "Use Dry Gas Meter?"() -> (w1590:bool)
            n740 = Array To Cluster(array=w1594) -> (cluster=w1593:T31)
            n741 = Unbundle(w1593) -> ("[0]"=w1592:dbl, "[1]"=→"Init Scale Temp":dbl, "[2]"=w1583:dbl, "[3]"=w1585:dbl, "[4]"=w1587:dbl, "[5]"=w1588:dbl)
            "WH_0" <- w1592
            n742 = case shown="True" w1590 {
              tunnel: [w1602 w1606] -> w1589
              tunnel: w1588 -> [_ w1606]
              tunnel: w1587 -> [_ w1605]
              tunnel: [w1602 w1605] -> w1586
              tunnel: w1585 -> [_ w1604]
              tunnel: [w1602 w1604] -> w1584
              tunnel: w1583 -> [_ w1603]
              tunnel: [w1602 w1603] -> w1582
              frame False {
                w1602 = 0.0 ("[2]")
              }
              frame True {
              }
            }
            n743 = call "E-Time.vi"() -> ("Elapsed Time (sec)"=w1598:dbl)  [unwired: 9 in, 2 out]
            "Start Time (sec)" <- w1598
            n744 = local read "2015?"() -> (w1581:bool)
            n745 = call "Worksheet DOE Audit.vi"() -> ("DOE Data Out"=w1600:T23)  [unwired: 8 in, 2 out]
            n746 = Bundle By Name(cluster=w1600, "Start Time(s)"=w1598, "Elect Energy Start"=w1592, "Gas Meter Pres"=w1582, "Gas Meter Temp"=w1584, "Barometer Pres"=w1586, "Gas Vol Init"=w1589) -> (w1599:T23)
            n747 = call "Worksheet DOE Audit.vi"("Add?"=TRUE, "DOE Data"=w1599, "2015?"=w1581) -> ()  [unwired: 5 in, 3 out]
          }
        }
        n748 = case shown="True" w1562 {
          tunnel: w1561 -> [_ w1580]
          frame False {
          }
          frame True {
            "Tend?" <- w1580
          }
        }
        n749 = Bundle By Name(cluster=w1572, "Enable RMC"=w1568) -> (w1571:T29)
        n750 = call <vilib>:"Add State(s) to Queue__jki_lib_state_machine.vi"("State(s) in Front (\"\")"="Data: Process Gas\nData: Process RMC", "State(s) in (\"\")"=w1579) -> ("States Out"=w1578:string)  [unwired: 13 in]
      }
      frame "Data: Process Gas" {
        # "If the current indicates the the dryer is on, go to the Data: Process RMC"
        n751 = Unbundle By Name(w1613) -> ("Q Element.Label Array"=w1615:string[], "Q Element.Data Array"=w1614:dbl[], "Power Previous"=w1612:bool)
        n752 = case shown="True" w1612 {
          tunnel: "Gas Pressure" ("Label") -> [_ w1629]
          tunnel: w1615 -> [_ w1628]
          tunnel: w1614 -> [_ w1626]
          frame False {
          }
          frame True {
            n753 = Search 1D Array(1D array=w1628, element=w1629) -> (index of element=w1627:i32)  [unwired: 1 in]
            n754 = Index Array(array=w1626, index=w1627) -> (element=w1625:dbl)
            n755 = while {
              tunnel: w1625 -> [w1633]
              shift-right: [w1631] -> _
              shift-left: _ -> [w1632]
              tunnel: [w1630] -> w1621
              stop <- TRUE stop-if-true
              n756 = Build Array (concatenate)(w1632, w1633) -> (w1631:dbl[])
              n757 = call-poly <vilib>:"Mean.vi"("X"=w1631) -> ("mean"=w1630:dbl)  [unwired: 1 out]
              "Ave Gas Pressure" <- w1630
            }
            n758 = call "Worksheet DOE Audit.vi"() -> ("DOE Data Out"=w1623:T23)  [unwired: 8 in, 2 out]
            n759 = Bundle By Name(cluster=w1623, "Gas Meter Pres"=w1621) -> (w1622:T23)
            n760 = local read "2015?"() -> (w1620:bool)
            n761 = call "Worksheet DOE Audit.vi"("Add?"=TRUE, "DOE Data"=w1622, "2015?"=w1620) -> ()  [unwired: 5 in, 3 out]
          }
        }
        n762 = call <vilib>:"Add State(s) to Queue__jki_lib_state_machine.vi"("State(s) in (\"\")"=w1619) -> ("States Out"=w1618:string)  [unwired: 14 in]